vi "HeartBeatDetectOffline2Breathing.vi"() -> ()   [LabVIEW 2014, in "Phonocardiography.lvlib"]
uses:
  Phonocardiography.lvlib
  <vilib>/Waveform/WDTOps.llb/WDT Index Channel DBL.vi
  <vilib>/Waveform/WDTOps.llb/WDT Get Waveform Time Array DBL.vi
  <vilib>/measure/NI_MABase.lvlib
  <vilib>/gmath/NI_Gmath.lvlib
panel:
  out "RR intervals Spectra":T1(graph)={"Power Spectrum FFT {X} Frequency"=[0.0, 0.008146511593538951, 0.016293023187077902, 0.024439534780616855, 0.032586046374155804, 0.04073255796769475, 0.04887906956123371, 0.05702558115477266, 0.06517209274831161, 0.07331860434185056, 0.0814651159353895, 0.08961162752892846, 0.09775813912246742, 0.10590465071600637, 0.11405116230954532, 0.12219767390308427, 0.13034418549662322, 0.13849069709016218, 0.14663720868370111, 0.15478372027724008, 0.162930231870779, 0.17107674346431798, 0.1792232550578569, 0.18736976665139587, 0.19551627824493484, 0.20366278983847377, 0.21180930143201274, 0.21995581302555167, 0.22810232461909064, 0.23624883621262957, 0.24439534780616853, 0.25254185939970747, 0.26068837099324643, 0.2688348825867854, 0.27698139418032436, 0.28512790577386327, 0.29327441736740223, 0.3014209289609412, 0.30956744055448016, 0.31771395214801906, 0.325860463741558, 0.334006975335097, 0.34215348692863595, 0.3502999985221749, 0.3584465101157138, 0.3665930217092528, 0.37473953330279175, 0.3828860448963307, 0.3910325564898697, 0.3991790680834086, 0.40732557967694755, 0.4154720912704865, 0.4236186028640255, 0.4317651144575644, 0.43991162605110334, 0.4480581376446423, 0.45620464923818127, 0.46435116083172023, 0.47249767242525914, 0.4806441840187981, 0.48879069561233707, 0.49693720720587603, 0.5050837187994149, 0.5132302303929539, 0.5213767419864929, 0.5295232535800318, 0.5376697651735708, 0.5458162767671098, 0.5539627883606487, 0.5621092999541876, 0.5702558115477265, 0.5784023231412655, 0.5865488347348045, 0.5946953463283434, 0.6028418579218824, 0.6109883695154213, 0.6191348811089603, 0.6272813927024993, 0.6354279042960381, 0.6435744158895771, 0.651720927483116, 0.659867439076655, 0.668013950670194, 0.6761604622637329, 0.6843069738572719, 0.6924534854508109, 0.7005999970443498, 0.7087465086378887, 0.7168930202314276, 0.7250395318249666, 0.7331860434185056, 0.7413325550120445, 0.7494790666055835, 0.7576255781991225, 0.7657720897926614, 0.7739186013862004, 0.7820651129797394, 0.7902116245732782, 0.7983581361668172, 0.8065046477603561, 0.8146511593538951, 0.8227976709474341, 0.830944182540973, 0.839090694134512, 0.847237205728051, 0.8553837173215899, 0.8635302289151288, 0.8716767405086677, 0.8798232521022067, 0.8879697636957457, 0.8961162752892846, 0.9042627868828236, 0.9124092984763625, 0.9205558100699015, 0.9287023216634405, 0.9368488332569793, 0.9449953448505183, 0.9531418564440572, 0.9612883680375962, 0.9694348796311352, 0.9775813912246741, 0.9857279028182131, 0.9938744144117521, 1.002020926005291, 1.0101674375988299, 1.018313949192369, 1.0264604607859078, 1.0346069723794469, 1.0427534839729857, 1.0508999955665246, 1.0590465071600637, 1.0671930187536025, 1.0753395303471416, 1.0834860419406804, 1.0916325535342195, 1.0997790651277584, 1.1079255767212974, 1.1160720883148363, 1.1242185999083751, 1.1323651115019142, 1.140511623095453, 1.1486581346889921, 1.156804646282531, 1.16495115787607, 1.173097669469609, 1.181244181063148, 1.1893906926566868], "Power Spectrum FFT {X}"=[1.2307762482654209e-25, 58.54413886193897, 233.13192484967468, 268.6004364109191, 99.73427477677255, 132.6024977717054, 182.06560795047446, 40.54399609526715, 88.49867269474333, 3.972996247494053, 28.791528739350905, 103.22397270634417, 196.88896248927418, 75.17737345421291, 45.34959450026026, 319.51553972495725, 140.0053099574313, 57.78425620106415, 47.55611510594588, 76.44699437715924, 67.95127090412481, 66.14069418100932, 101.92152768682767, 164.90842663611127, 73.59023836375823, 13.249589339821283, 53.2134874317107, 96.28393773444884, 131.37865367113724, 234.5673928825604, 276.1893823008717, 242.78368684558563, 20.58774975515059, 47.541104319174224, 96.79332290607519, 35.716179335141426, 43.796769374212666, 68.71449011042318, 22.879276333439808, 11.18192779529983, 50.064944393829606, 6.270246825768338, 0.2625027883484574, 2.0499963059394224, 3.752228673935682, 9.961226604065034, 6.443787839885471, 0.4711467652802496, 1.0757126983749261, 0.635121350373348, 1.8151342605051741, 5.302704636907321, 1.1432295739121592, 4.702947979708913, 4.321724461579127, 4.630878048479111, 5.146522558120115, 10.33903278698432, 5.849563625491225, 0.743868020259558, 1.933625998634512, 4.244931480200766, 9.205542268517291, 3.866486311407042, 3.368229735182078, 1.6964207204669655, 4.55801194485727, 2.1030986302130454, 3.426801712346284, 3.364280599305024, 0.09951564768032004, 1.5777595891933012, 5.039739268674444, 4.066037233949989, 2.582064061304811, 8.32390405571162, 10.947686376494753, 9.37032306678097, 15.54957291286616, 25.45959178545612, 1.1259355678763159, 14.625045821415181, 16.07182002806382, 3.3049306634400244, 4.4803245487316, 2.2984024147472812, 1.9869917591666162, 0.8588879907961221, 9.859289365719182, 18.30275715466448, 9.702851589139177, 2.448152713757161, 10.496223901449566, 10.700812590422155, 4.242793063562076, 7.68671894750528, 40.138943788129936, 101.43859983643893, 2.724792836691798, 23.099133368616542, 18.199597167490438, 10.453380912262785, 0.6161661011064901, 1.4971595857081408, 0.6424508334667665, 29.446527845270758, 30.634564689919966, 1.5672037628411288, 17.04963861636795, 47.29180351271122, 11.626489853787795, 208.85672456415895, 278.00127178575735, 12.510124780376087, 37.90380488369466, 27.64871897870445, 80.72648777589632, 2.6048168152883164, 76.50452952187149, 13.357416307301724, 36.6687515067713, 35.32469555604035, 142.12390637748348, 20.5759948502237, 31.96796012612855, 34.49661937547406, 111.96815819529613, 1.1103644076541908, 189.8799865307011, 34.28340849477395, 26.02035215999174, 51.71237124661553, 30.86489975380715, 2.024137726683583, 41.30928004344402, 4.266977524160255, 5.031048883138152, 3.4195096308248796, 10.057449627151751, 42.910483346908755, 39.28326968142908, 168.40845644164386, 16.283948755416233, 100.72635339166334, 6.488017871388993, 3.1629278803688936, 1.8698285176664373]}
  in  "Remove\nEctopic Beats":bool=TRUE
  out "pNN50 [%]":dbl=21.232876712328768 format="%.1f"
  out "rMSSD  [ms] 2":dbl=68.85967760569123
  out "sdRR [ms]":dbl=81.8447364744125
  out "Mean RR [ms]":dbl=843.4299467994049 format="%_1f"
  out "Mean heart rate [BPM]":dbl=71.13809537790807 format="%#.1g"
  in  "Negate":bool
  out "Heart rate":T2(graph)=[{"X [s]"=[1.0717460317460312, 1.80517006802721, 2.5313378684807244, 3.290975056689341, 4.021224489795917, 4.70439909297052, 5.478639455782311, 6.424126984126981, 7.393197278911561, 7.796190476190473, 8.327437641723353, 8.847437641723353, 9.405170068027207, 9.964353741496595, 10.772154195011334, 11.603537414965981, 12.395011337868475, 13.184852607709745, 14.145306122448973, 15.155192743764166, 16.14068027210884, 17.033469387755094, 17.822131519274368, 18.64335600907029, 19.487619047619038, 20.375328798185933, 21.22839002267573, 22.09015873015872, 23.05795918367346, 24.05832199546484, 24.99410430839001, 25.799637188208607, 26.6073469387755, 27.47473922902493, 28.39437641723355, 29.231383219954637, 29.97877551020407, 30.762539682539668, 31.684172335600895, 32.67800453514738, 33.57396825396824, 34.4517006802721, 35.36925170068026, 36.28861678004534, 37.15555555555554, 37.95655328798184, 38.77551020408161, 39.65396825396824, 40.55764172335599, 41.41306122448978, 42.231564625850325, 43.0978684807256, 43.9931065759637, 44.85678004535146, 45.67555555555553, 46.53306122448978, 47.4449886621315, 48.34476190476188, 49.17569160997731, 49.996462585033996, 50.84081632653059, 51.72117913832197, 52.59909297052152, 53.41514739229023, 54.19619047619045, 55.033197278911544, 55.98503401360542, 56.90684807256233, 57.75981859410428, 58.61931972789113, 59.50086167800451, 60.36961451247163, 61.17061224489793, 61.92444444444442, 62.72108843537412, 63.64117913832197, 64.58993197278909, 65.45814058956913, 66.26476190476188, 67.12761904761902, 67.99945578231289, 68.84235827664396, 69.60662131519271, 70.34802721088433, 71.14340136054419, 72.01424036281176, 72.89895691609975, 73.7321541950113, 74.63265306122446, 75.49950113378682, 76.35229024943307, 77.16163265306119, 77.9244444444444, 78.7406802721088, 79.62376417233557, 80.51482993197276, 81.34285714285711, 82.16371882086165, 82.98585034013603, 83.80099773242627, 84.58294784580495, 85.30902494331062, 86.04371882086164, 86.8790929705215, 87.71265306122446, 88.51310657596368, 89.29442176870745, 90.11845804988658, 91.04770975056685, 91.951746031746, 92.83129251700676, 93.60943310657592, 94.33342403628114, 95.11464852607706, 96.10811791383216, 97.0424489795918, 97.87301587301583, 98.73560090702944, 99.6119727891156, 100.47990929705212, 101.28988662131515, 102.05941043083895, 102.92235827664395, 103.86539682539679, 104.79102040816322, 105.62947845804985, 106.49442176870744, 107.41741496598635, 108.33024943310653, 109.14539682539677, 109.91655328798181, 110.7006802721088, 111.55909297052149, 112.48725623582762, 113.36698412698408, 114.20988662131515, 115.1309750566893, 116.04380952380947, 116.96145124716548, 117.8107936507936, 118.61242630385482, 119.44879818594099, 120.3123809523809, 121.14938775510198, 121.9503854875283, 122.88353741496593, 123.8236734693877], "Heart Rate [BPM]"=[70.17078604009762, 81.80806331931737, 82.62553085186114, 78.98507462686567, 82.1637063718793, 87.82527881040896, 77.49531396438616, 63.4593246354567, 61.9150131037065, 76.9022492495641, 112.94177906778204, 115.38461538461549, 107.57846804358446, 107.2992700729927, 74.27576914439706, 72.16888500981902, 75.80793032317217, 75.96463022508034, 62.47048824251586, 59.41261002335189, 60.88357109986189, 67.20512039012517, 76.07820586543993, 73.06163021868771, 71.06789858186532, 67.5896597527331, 70.33492822966507, 69.62425007893924, 61.996251171508796, 59.978239187596536, 64.11747601046817, 74.48485530908663, 74.28411005053344, 69.17285370699592, 65.24312062333553, 71.68400520156047, 80.27912621359225, 76.55363962504369, 65.1018600531442, 60.37236469836633, 66.96699736788844, 68.35796217836082, 65.39145907473319, 65.26243093922655, 69.20903954802297, 74.90657909636512, 73.26392734522106, 68.30149716055729, 66.39566395663958, 70.14102428162433, 73.30452127659571, 69.25976337556331, 67.02127659574438, 69.4706994328922, 73.28015952143613, 69.97038290670581, 65.79470857370208, 66.6834677419358, 72.20827420587224, 73.10200022101891, 71.06026426039328, 68.15371934885671, 68.34383717326173, 73.5245081693894, 76.82034606898198, 71.68400520156017, 63.03602058319041, 65.08904850929875, 70.34240748617624, 69.80793583790614, 68.0625578763246, 69.06452286489902, 74.90657909636512, 79.59331007099007, 75.31595126949817, 65.21096214511041, 63.240917782026656, 69.10781445883887, 74.38434723940055, 69.53642384106003, 68.82022471910156, 71.18261056709309, 78.50700213624546, 80.92733056031278, 75.43619568936026, 68.89907301322785, 67.81833094115196, 72.01175702155534, 66.62973408541474, 69.21628125980924, 70.35737077217718, 74.13425977810115, 78.65636147443578, 73.50816757417483, 67.94371405094435, 67.33509771986985, 72.46138678935228, 73.09392265193387, 72.98102383053818, 73.60632024034778, 76.73123767544372, 82.63585259213028, 81.66666666666627, 71.82410423452838, 71.98041349292603, 74.95750708215405, 76.7935918272568, 72.81232801320907, 64.5680819912155, 66.36901775860288, 68.21697432195603, 77.10688891479184, 82.87396642445408, 76.80250783699069, 60.39441248972906, 64.21706630424238, 72.23981653379944, 69.5583596214511, 68.46408611053663, 69.12948061448333, 74.07614781635012, 77.97029702970353, 69.5291149884375, 63.62412234298329, 64.82116609505185, 71.55993076590184, 69.36870805369146, 65.00589622641498, 65.72933227345021, 73.60632024034778, 77.80522230063454, 76.5182186234817, 69.8964497041425, 64.64379947229533, 68.20290751623874, 71.18261056709309, 65.14032496307271, 65.72933227345021, 65.38499555204083, 70.64288765484868, 74.84725050916548, 71.73842316451567, 69.47799600882185, 71.68400520156138, 74.90657909636447, 64.29821150855413, 63.82054992764095]}, {"X [s]"=array[1368064 elements], "Heart Rate [BPM]"=array[1368064 elements]}]
  out "Heart beats":cluster{"Peaks X":dbl[], "Peaks Y":dbl[]}[](graph)=[{"Peaks X"=array[1368064 elements], "Peaks Y"=array[1368064 elements]}, {"Peaks X"=[0.21668934240362803, 1.0717460317460312, 1.80517006802721, 2.5313378684807244, 3.290975056689341, 4.021224489795917, 4.70439909297052, 5.478639455782311, 6.424126984126981, 7.393197278911561, 7.796190476190473, 8.327437641723353, 8.847437641723353, 9.405170068027207, 9.964353741496595, 10.772154195011334, 11.603537414965981, 12.395011337868475, 13.184852607709745, 14.145306122448973, 15.155192743764166, 16.14068027210884, 17.033469387755094, 17.822131519274368, 18.64335600907029, 19.487619047619038, 20.375328798185933, 21.22839002267573, 22.09015873015872, 23.05795918367346, 24.05832199546484, 24.99410430839001, 25.799637188208607, 26.6073469387755, 27.47473922902493, 28.39437641723355, 29.231383219954637, 29.97877551020407, 30.762539682539668, 31.684172335600895, 32.67800453514738, 33.57396825396824, 34.4517006802721, 35.36925170068026, 36.28861678004534, 37.15555555555554, 37.95655328798184, 38.77551020408161, 39.65396825396824, 40.55764172335599, 41.41306122448978, 42.231564625850325, 43.0978684807256, 43.9931065759637, 44.85678004535146, 45.67555555555553, 46.53306122448978, 47.4449886621315, 48.34476190476188, 49.17569160997731, 49.996462585033996, 50.84081632653059, 51.72117913832197, 52.59909297052152, 53.41514739229023, 54.19619047619045, 55.033197278911544, 55.98503401360542, 56.90684807256233, 57.75981859410428, 58.61931972789113, 59.50086167800451, 60.36961451247163, 61.17061224489793, 61.92444444444442, 62.72108843537412, 63.64117913832197, 64.58993197278909, 65.45814058956913, 66.26476190476188, 67.12761904761902, 67.99945578231289, 68.84235827664396, 69.60662131519271, 70.34802721088433, 71.14340136054419, 72.01424036281176, 72.89895691609975, 73.7321541950113, 74.63265306122446, 75.49950113378682, 76.35229024943307, 77.16163265306119, 77.9244444444444, 78.7406802721088, 79.62376417233557, 80.51482993197276, 81.34285714285711, 82.16371882086165, 82.98585034013603, 83.80099773242627, 84.58294784580495, 85.30902494331062, 86.04371882086164, 86.8790929705215, 87.71265306122446, 88.51310657596368, 89.29442176870745, 90.11845804988658, 91.04770975056685, 91.951746031746, 92.83129251700676, 93.60943310657592, 94.33342403628114, 95.11464852607706, 96.10811791383216, 97.0424489795918, 97.87301587301583, 98.73560090702944, 99.6119727891156, 100.47990929705212, 101.28988662131515, 102.05941043083895, 102.92235827664395, 103.86539682539679, 104.79102040816322, 105.62947845804985, 106.49442176870744, 107.41741496598635, 108.33024943310653, 109.14539682539677, 109.91655328798181, 110.7006802721088, 111.55909297052149, 112.48725623582762, 113.36698412698408, 114.20988662131515, 115.1309750566893, 116.04380952380947, 116.96145124716548, 117.8107936507936, 118.61242630385482, 119.44879818594099, 120.3123809523809, 121.14938775510198, 121.9503854875283, 122.88353741496593, 123.8236734693877], "Peaks Y"=[0.201629638671875, 0.192962646484375, 0.213836669921875, 0.209014892578125, 0.205413818359375, 0.18658447265625, 0.20831298828125, 0.272430419921875, 0.238372802734375, 0.219329833984375, 0.125732421875, 0.18994140625, 0.128082275390625, 0.09893798828125, 0.183624267578125, 0.169097900390625, 0.19970703125, 0.200042724609375, 0.220733642578125, 0.21014404296875, 0.22100830078125, 0.17681884765625, 0.207855224609375, 0.21734619140625, 0.164459228515625, 0.166290283203125, 0.189208984375, 0.193267822265625, 0.1942138671875, 0.163330078125, 0.218475341796875, 0.165557861328125, 0.157012939453125, 0.152130126953125, 0.137481689453125, 0.184234619140625, 0.1441650390625, 0.166717529296875, 0.128570556640625, 0.168548583984375, 0.168731689453125, 0.149444580078125, 0.14691162109375, 0.1910400390625, 0.15167236328125, 0.13525390625, 0.175018310546875, 0.123992919921875, 0.168548583984375, 0.15008544921875, 0.141387939453125, 0.139434814453125, 0.14385986328125, 0.151214599609375, 0.151275634765625, 0.166107177734375, 0.11834716796875, 0.174407958984375, 0.137786865234375, 0.151580810546875, 0.13751220703125, 0.139801025390625, 0.17926025390625, 0.14227294921875, 0.141571044921875, 0.14837646484375, 0.13397216796875, 0.186920166015625, 0.125518798828125, 0.149078369140625, 0.15155029296875, 0.15460205078125, 0.1619873046875, 0.116912841796875, 0.1724853515625, 0.12261962890625, 0.166290283203125, 0.150177001953125, 0.148468017578125, 0.18017578125, 0.120941162109375, 0.151336669921875, 0.158203125, 0.1790771484375, 0.137786865234375, 0.156158447265625, 0.166778564453125, 0.147857666015625, 0.17822265625, 0.1409912109375, 0.143402099609375, 0.159912109375, 0.14312744140625, 0.17120361328125, 0.1217041015625, 0.15777587890625, 0.148040771484375, 0.17626953125, 0.146087646484375, 0.119842529296875, 0.1455078125, 0.134796142578125, 0.153167724609375, 0.155242919921875, 0.149688720703125, 0.152496337890625, 0.16204833984375, 0.188507080078125, 0.146392822265625, 0.1685791015625, 0.17132568359375, 0.12103271484375, 0.1685791015625, 0.154754638671875, 0.14630126953125, 0.1690673828125, 0.1383056640625, 0.16705322265625, 0.126739501953125, 0.16619873046875, 0.13958740234375, 0.1534423828125, 0.144744873046875, 0.1336669921875, 0.157562255859375, 0.1373291015625, 0.16473388671875, 0.1514892578125, 0.15313720703125, 0.13812255859375, 0.1527099609375, 0.17401123046875, 0.150604248046875, 0.1429443359375, 0.15435791015625, 0.147735595703125, 0.1685791015625, 0.146759033203125, 0.157257080078125, 0.150054931640625, 0.152862548828125, 0.13958740234375, 0.13262939453125, 0.1474609375, 0.147857666015625, 0.157257080078125, 0.140716552734375, 0.164642333984375]}]
  in  "Max time to peak\nfrom threshold (ms)":dbl=150.0
  in  "Threshold mult 2":dbl=0.35 min=-1.0 max=1.0 step=0.05
  in  "Min time between\nbeats (ms)":dbl=400.0
  in  "width (threshold) 2":i32=3
  in  "File Path Control":path=path "C:/Users/Tamas/Documents/Projektek/Szívhang/Felvételek cikkhez/breath_3.wav"
  in  "Breathing freq \n[1/min]":dbl=15.0
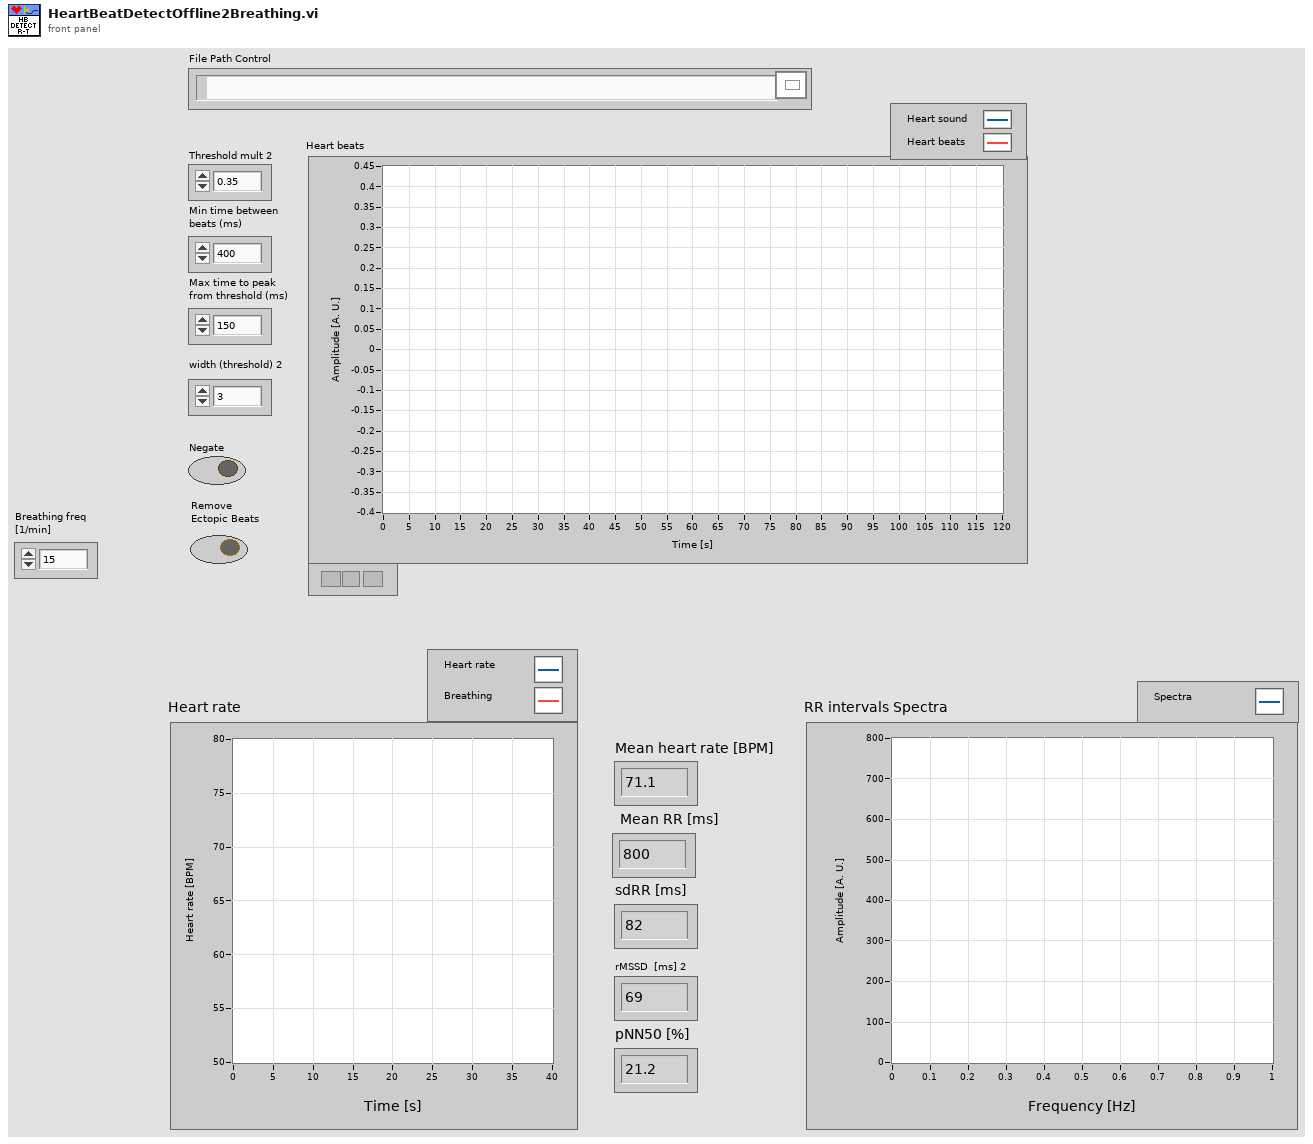
[diagram p1: front panel]
types:
  T1 = cluster{"Power Spectrum FFT {X} Frequency":dbl[], "Power Spectrum FFT {X}":dbl[]}
  T2 = cluster{"X [s]":dbl[], "Heart Rate [BPM]":dbl[]}[]
  T3 = typedef "LVCursorListTypeDef.ctl" = cluster{"Name":string, "Color":u32, "Style":u8, "Point Style":u8, "Name Visible":bool, "Allow Drag":bool, "Cursor Mode":u32, "Plot":i32, "Index":i32, "Position":cluster{"X":dbl, "Y":dbl}, "X Scale":u32, "Y Scale":u32, "Watch Plots":i32[], "Watch All Plots":bool, "Plot Area":i32, "Label Offset":cluster{"X":dbl, "Y":dbl}}[]
  T4 = cluster{"Name":string, "Color":u32, "Style":u8, "Point Style":u8, "Name Visible":bool, "Allow Drag":bool, "Cursor Mode":u32, "Plot":i32, "Index":i32, "Position":cluster{"X":dbl, "Y":dbl}, "X Scale":u32, "Y Scale":u32, "Watch Plots":i32[], "Watch All Plots":bool, "Plot Area":i32, "Label Offset":cluster{"X":dbl, "Y":dbl}}
  T5 = cluster{"Name":string, "Color":u32, "Style":u8, "Point Style":u8, "Name Visible":bool, "Allow Drag":bool, "Cursor Mode":u32, "Plot":i32, "Index":i32, "Position":cluster{"X":dbl, "Y":dbl}, "X Scale":u32, "Y Scale":u32, "Watch Plots":i32[], "Watch All Plots":bool, "Plot Area":i32, "Label Offset":cluster{"X":dbl, "Y":dbl}}[]
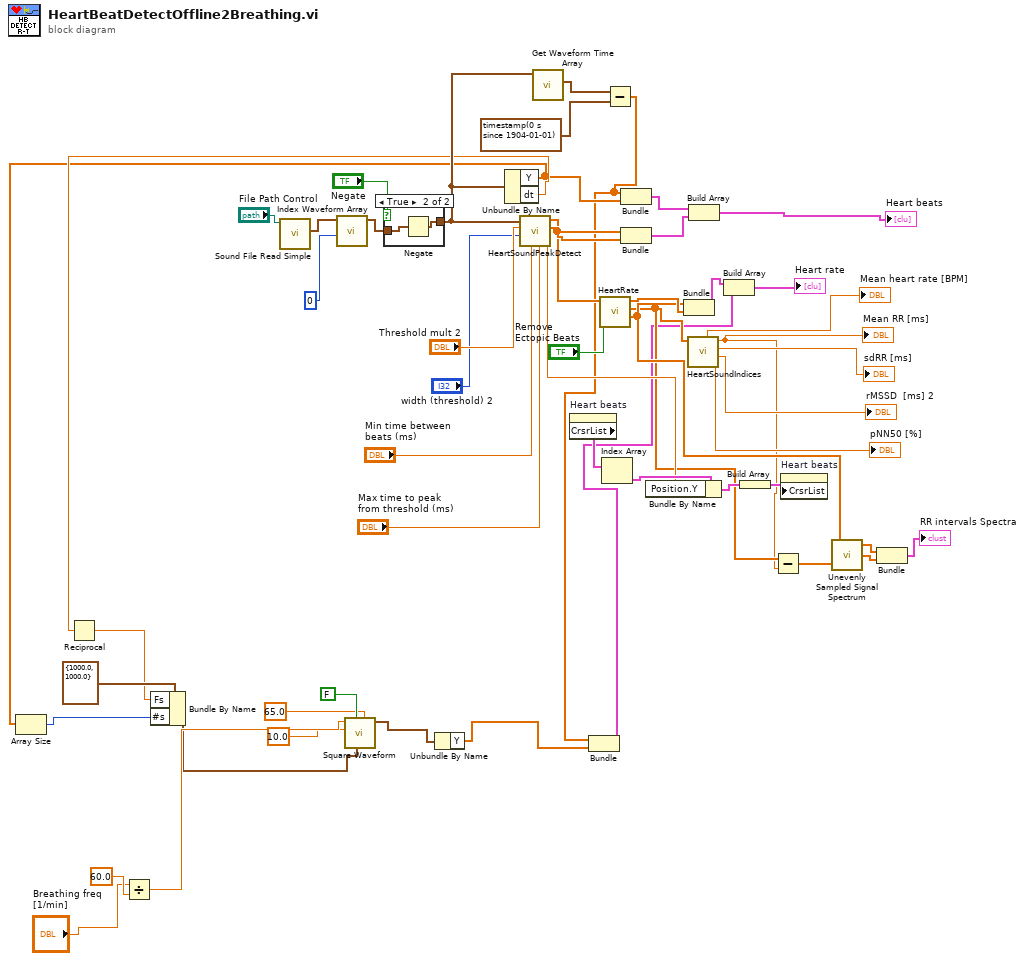
[diagram p0: block diagram]
diagram:
  n1 = Divide(x="Breathing freq \n[1/min]", y=60.0) -> (x/y=w52:dbl)
  n2 = call <vilib>:"Sound File Read Simple.vi"("path"="File Path Control") -> ("data"=w47:waveform(dbl)[])  [unwired: 7 in, 3 out]
  n3 = call-poly <vilib>:"Index Waveform Array.vi"("index"=0, "waveform array"=w47) -> ("waveform"=w28:waveform(dbl))  [unwired: 8 in, 1 out]
  n4 = case shown="True" "Negate" {
    tunnel: w28 -> [w54 w56]
    tunnel: [w54 w55] -> w27
    frame False {
    }
    frame True {
      n5 = Negate(x=w56) -> (-x=w55:waveform(dbl))
    }
  }
  n6 = Unbundle By Name(w27) -> ("Y"=w9:dbl[], "dt"=w10:dbl)
  n7 = Array Size(array=w9) -> (size(s)=w8:i32)
  n8 = Reciprocal(x=w10) -> (1/x=w3:dbl)
  n9 = Bundle By Name(cluster=cluster{"Fs":dbl, "#s":dbl} {"Fs"=1000.0, "#s"=1000.0} ("sampling info"), "Fs"=w3, "#s"=w8) -> (w50:cluster{"Fs":dbl, "#s":dbl})
  n10 = call <vilib>:"Square Waveform.vi"("offset"=65.0 ("amplitude"), "sampling info"=w50, "reset signal"=FALSE, "amplitude"=10.0, "frequency"=w52) -> ("signal out"=w12:waveform(dbl))  [unwired: 5 in, 1 out]
  n11 = Unbundle By Name(w12) -> ("Y"=w2:dbl[])
  n12 = call "HeartSoundPeakDetect.vi"("Max time to peak\nfrom threshold (ms)"="Max time to peak\nfrom threshold (ms)", "Min time between\nbeats (ms)"="Min time between\nbeats (ms)", "width (threshold)"="width (threshold) 2", "Threshold multiplier"="Threshold mult 2", "Sound"=w27) -> ("Threshold"=w29:dbl, "Peaks Y"=w41:dbl[], "Peaks X"=w38:dbl[])  [unwired: 4 in]
  n13 = call-poly <vilib>:"Get Waveform Time Array.vi"("waveform in"=w27) -> ("X array"=w36:timestamp[])  [unwired: 9 in, 1 out]
  n14 = property on="Heart beats" class="XYGraph (strict)"() -> ("CrsrList"=w31:T3)  [unwired: 2 in, 2 out]
  n15 = call "HeartRate.vi"("Remove Ectopic?"="Remove\nEctopic Beats", "Peaks X in"=w38) -> ("X [s]"=w20:dbl[], "RR intervals [ms]"=w15:dbl[], "Heart Rate [BPM]"=w37:dbl[])  [unwired: 7 in]
  n16 = Index Array(array=w31) -> (element=w33:T4)  [unwired: 1 in]
  n17 = Subtract(x=w36, y=timestamp(0 s since 1904-01-01) ("Xo")) -> (x-y=w7:dbl[])
  n18 = Bundle(w7, "Y"=w2) -> (w5:cluster{dbl[], "Y":dbl[]})  [unwired: 1 in]
  n19 = Bundle(w7, "Y"=w9) -> (w40:cluster{dbl[], "Y":dbl[]})  [unwired: 1 in]
  n20 = Bundle("Peaks X"=w38, "Peaks Y"=w41) -> (w39:cluster{"Peaks X":dbl[], "Peaks Y":dbl[]})  [unwired: 1 in]
  n21 = Bundle By Name(cluster=w33, "Position.Y"=w29) -> (w32:T4)
  n22 = Bundle("X [s]"=w20, "Heart Rate [BPM]"=w37) -> (w6:cluster{"X [s]":dbl[], "Heart Rate [BPM]":dbl[]})  [unwired: 1 in]
  n23 = call "HeartSoundIndices.vi"("RR intervals [ms]"=w15) -> ("pNN50 [%]"=→"pNN50 [%]":dbl, "rMSSD  [ms]"=→"rMSSD  [ms] 2":dbl, "sdRR [ms]"=→"sdRR [ms]":dbl, "Mean RR [ms]"=w14:dbl, "Mean heart rate [BPM]"=→"Mean heart rate [BPM]":dbl)  [unwired: 6 in]
  "Mean RR [ms]" <- w14
  n24 = Build Array(w40, w39) -> (→"Heart beats":cluster{"Peaks X":dbl[], "Peaks Y":dbl[]}[])
  n25 = Build Array(w6, w5) -> (→"Heart rate":cluster{"X [s]":dbl[], "Y":dbl[]}[])
  n26 = Build Array(w32) -> (w30:T5)
  n27 = Subtract(x=w15, y=w14) -> (x-y=w16:dbl[])
  n28 = property on="Heart beats" class="XYGraph (strict)"("CrsrList"=w30) -> ()  [unwired: 2 in, 2 out]
  n29 = call <vilib>:"Unevenly Sampled Signal Spectrum.vi"("XTime"=w20, "X"=w16) -> ("Power Spectrum FFT {X} Frequency"=w19:dbl[], "Power Spectrum FFT {X}"=w18:dbl[])  [unwired: 1 out]
  n30 = Bundle("Power Spectrum FFT {X} Frequency"=w19, "Power Spectrum FFT {X}"=w18) -> (→"RR intervals Spectra":T1)  [unwired: 1 in]
